vi "UHR-Fleezers Control (host) - 12.3.1.vi"() -> ()   [LabVIEW 2012] (continued)
              }
            }
          }
          frame #3 {
            n739 = property on="Sample Channel\nFlow" class="Bool (strict)"("Val(Sgnl)"=FALSE ("Value (Signaling)")) -> ()  [unwired: 2 in, 2 out]
            n740 = case shown="False" "Cap. 2 BD T1?\n(ADig T1, DNA T2)" {
              tunnel: "Cap 2 T ON" -> [w1060 w1061]
              frame False {
                n741 = property on="Trap 2 (ON/OFF)" class="Bool (strict)"("Val(Sgnl)"=w1060) -> ()  [unwired: 2 in, 2 out]
              }
              frame True {
                n742 = property on="Trap 1 (ON/OFF)" class="Bool (strict)"("Val(Sgnl)"=w1061) -> ()  [unwired: 2 in, 2 out]
              }
            }
            n743 = property on="Got ADig bead" class="Bool"("Key Focus"=TRUE) -> ()  [unwired: 2 in, 2 out]
          }
        }
      }
      event "Read Harvard": Value Change {
        n744 = event-data() -> ()  [unwired: 1 in, 5 out]
        n745 = Concatenate Strings("write buffer", "\r") -> (w1066:string)
        n746 = VISA Write(VISA resource name=w1064, write buffer=w1066, error in (no error)=w1063) -> (VISA resource name out=w1075:refnum<visa-resource-name>, error out=w1074:errorcluster)  [unwired: 1 out]
        n747 = stacked-sequence {
          tunnel: [w1078] -> w1073
          tunnel: w1075 -> [w1078]
          tunnel: w1074 -> [w1077]
          tunnel: [w1077] -> w1068
          frame #0 {
            n748 = Wait (ms)(milliseconds to wait=50) -> ()  [unwired: 1 out]
          }
        }
        n749 = property class="Instr"(reference=w1073, error in=w1068) -> (reference out=w1072:refnum<visa-resource-name>, error out=w1070:errorcluster, "Serial Settings:Number of Bytes at Serial Port"=w1071:u32)
        "Serial Settings:Number of Bytes at Serial Port" <- w1071
        n750 = VISA Read(VISA resource name=w1072, byte count=w1071, error in (no error)=w1070) -> (read buffer=w1069:string)  [unwired: 3 out]
        "read buffer" <- w1069
        n751 = Fract/Exp String To Number(string=w1069) -> ()  [unwired: 5 out]
      }
      event "+z", "-z": Value Change {
        n752 = event-data() -> ()  [unwired: 1 in, 5 out]
        n753 = flat-sequence {
          tunnel: w1079 -> [w1101]
          tunnel: w1080 -> [w1081]
          frame #0 {
            n754 = call "Read Stage Position.vi"("error in"=w1101, "VISA resource name in"=w1081) -> ("Current Position"=w1086:cluster{dbl, dbl, dbl}, "error out"=w1099:errorcluster, "VISA resource name out"=w1100:refnum<visa-resource-name>)  [unwired: 1 out]
            n755 = local read "Saved Stage Positions"() -> (w1110:dbl[][])
            n756 = Divide(x="z nudge increment (um)", y=1000.0) -> (x/y=w1098:dbl)
            n757 = Boolean To (0,1)(Boolean="+z") -> (0, 1=w1090:i16)
            n758 = Boolean To (0,1)(Boolean="-z") -> (0, 1=w1091:i16)
            n759 = Array Subset(array=w1110, index (row)=1 ("index"), length (row)=1 ("length"), index (col)=1 ("index"), length (col)=3 ("length")) -> (w1107:dbl[][])
            n760 = Multiply(x=w1090, y=w1098) -> (x*y=w1094:dbl)
            n761 = Multiply(x=w1091, y=w1098) -> (x*y=w1092:dbl)
            n762 = Unbundle(w1086) -> (w1084:dbl, w1083:dbl, w1087:dbl)
            n763 = Negate(x=w1092) -> (-x=w1093:dbl)
            n764 = Reshape Array(w1107, 3 ("dimension size")) -> (w1105:dbl[])
            n765 = Add(x=w1094, y=w1093) -> (x+y=w1095:dbl)
            n766 = Array To Cluster(array=w1105) -> ()  [unwired: 1 out]
            n767 = Add(x=w1095, y=w1087) -> (x+y=w1085:dbl)
            n768 = Bundle(cluster=w1086, w1084, w1083, w1085) -> (w1082:cluster{dbl, dbl, dbl})
            n769 = call "Set Stage Position.vi"("Position"=w1082, "error in"=w1099, "VISA resource name in"=w1100) -> ("error out"=w1104:errorcluster)  [unwired: 2 out]
            n770 = local write "Stage Moving"(TRUE ("Stage Moving")) -> ()
            n771 = local write "Stage Control Serial Error"(w1104) -> ()
          }
          frame #1 {
            n772 = local write "Stage Moving"(FALSE ("Stage Moving")) -> ()
            n773 = call <vilib>:"Beep.vi"() -> ()  [unwired: 3 in, 9 out]
          }
        }
      }
      event "Cal/Data Acq. Spot": Value Change {
        n774 = event-data() -> ()  [unwired: 1 in, 5 out]
        n775 = flat-sequence {
          tunnel: w1119 -> [w1123]
          tunnel: w1120 -> [w1124]
          tunnel: [w1124] -> w1116
          tunnel: [w1123] -> w1115
          tunnel: w1116 -> [w1129]
          tunnel: w1115 -> [w1128]
          tunnel: ["Cal @ (MHz)"] -> w1113
          tunnel: [w1133] -> w1117
          tunnel: w1113 -> [w1133]
          tunnel: w1117 -> [w1142]
          tunnel: ["W/ Offset 1"] -> w1114
          tunnel: w1117 -> [w1163]
          tunnel: w1114 -> [w1161]
          frame #0 {
            n776 = property on="Sample Channel\nFlow" class="Bool (strict)"("Val(Sgnl)"="Daq spot flow on") -> ()  [unwired: 2 in, 2 out]
            n777 = Wait (ms)(milliseconds to wait=u32 250) -> ()  [unwired: 1 out]
          }
          frame #1 {
            n778 = local read "Saved Stage Positions"() -> (w1126:dbl[][])
            n779 = property on="Trap Delta (MHz)" class="DigNum (strict)"("Val(Sgnl)"="Cal @ (MHz)") -> ()  [unwired: 2 in, 2 out]
            n780 = local write "Stage Moving"(TRUE ("Stage Moving")) -> ()
            n781 = call "move to saved stage position.vi"("error in"=w1128, "Stage VISA resource name in"=w1129, "Position"="Cal Stage Position", "Saved Stage Positions"=w1126) -> ("error out"=w1127:errorcluster)  [unwired: 1 out]
            n782 = local write "Stage Control Serial Error"(w1127) -> ()
          }
          frame #2 {
            n783 = local write "Stage Moving"(FALSE ("Stage Moving")) -> ()
            n784 = property on="Sample Channel\nFlow" class="Bool (strict)"("Val(Sgnl)"="Flow ON during cal?") -> ()  [unwired: 2 in, 2 out]
            n785 = call <vilib>:"Beep.vi"() -> ()  [unwired: 3 in, 9 out]
          }
          frame #3 {
            n786 = Wait (ms)(milliseconds to wait=u32 1000) -> ()  [unwired: 1 out]
          }
          frame #4 {
            n787 = property on="Save Calibration" class="Bool (strict)"("Val(Sgnl)"=TRUE ("Value (Signaling)")) -> ()  [unwired: 2 in, 2 out]
          }
          frame #5 {
            n788 = Wait (ms)(milliseconds to wait=u32 2000) -> ()  [unwired: 1 out]
          }
          frame #6 {
            # "Check to see if \nsaving done"
            n789 = while {
              stop <- w1138 stop-if-true
              n790 = local read "Saving..."() -> (w1139:bool)
              n791 = Wait (ms)(milliseconds to wait=u32 100) -> ()  [unwired: 1 out]
              n792 = Not(x=w1139) -> (.not. x?=w1138:bool)
            }
          }
          frame #7 {
            n793 = case shown="True" "W/ Offset 1" {
              tunnel: w1142 -> [_ w1143]
              frame False {
              }
              frame True {
                n794 = stacked-sequence {
                  tunnel: w1143 -> [_ _ _ _ _ _ _ w1160]
                  frame #0 {
                    n795 = property on="Trap Delta (MHz)" class="DigNum (strict)"("Val(Sgnl)"="Offset 1 Start (MHz)") -> ()  [unwired: 2 in, 2 out]
                    n796 = Replace Array Subset(array=u32[] [0] ("Index Values"), new element="Offset 1 Set", index=0) -> (w1144:u32[])
                    n797 = property on="Saved AOD Raster Scan Parameter Sets" class="Arr (strict)"("Index Values"=w1144) -> ()  [unwired: 2 in, 2 out]
                  }
                  frame #1 {
                    n798 = Wait (ms)(milliseconds to wait=u32 200) -> ()  [unwired: 1 out]
                  }
                  frame #2 {
                    n799 = property on="Load parameters" class="Bool (strict)"("Val(Sgnl)"=TRUE ("Value (Signaling)")) -> ()  [unwired: 2 in, 2 out]
                  }
                  frame #3 {
                    n800 = Wait (ms)(milliseconds to wait=u32 200) -> ()  [unwired: 1 out]
                  }
                  frame #4 {
                    n801 = property on="Trap Raster Scan" class="Bool (strict)"("Val(Sgnl)"=TRUE ("Value (Signaling)")) -> ()  [unwired: 2 in, 2 out]
                  }
                  frame #5 {
                    n802 = Wait (ms)(milliseconds to wait=u32 2000) -> ()  [unwired: 1 out]
                  }
                  frame #6 {
                    n803 = while {
                      stop <- w1157 stop-if-true
                      n804 = local read "Raster Scanning..."() -> (w1159:bool)
                      n805 = local read "Saving..."() -> (w1155:bool)
                      n806 = Wait (ms)(milliseconds to wait=u32 100) -> ()  [unwired: 1 out]
                      n807 = Not(x=w1155) -> (.not. x?=w1154:bool)
                      n808 = Not(x=w1159) -> (.not. x?=w1156:bool)
                      n809 = And(x=w1156, y=w1154) -> (x .and. y?=w1157:bool)
                    }
                  }
                  frame #7 {
                    n810 = property on="Trap Delta (MHz)" class="DigNum (strict)"("Val(Sgnl)"=w1160) -> ()  [unwired: 2 in, 2 out]
                  }
                }
              }
            }
          }
          frame #8 {
            n811 = local read "Save ave N"() -> (w1162:dbl)
            n812 = case shown="False" "W/ Offset 2" {
              tunnel: w1163 -> [_ w1170]
              tunnel: w1162 -> [_ w1169]
              tunnel: w1161 -> [w1165 _]
              frame False {
                n813 = case shown="False" w1165 {
                  frame False {
                    n814 = Multiply(x="Cal read wait (s)", y=u32 1000 ("milliseconds to wait")) -> (x*y=w1167:u32)
                    n815 = Wait (ms)(milliseconds to wait=w1167) -> ()  [unwired: 1 out]
                  }
                  frame True {
                  }
                }
              }
              frame True {
                n816 = stacked-sequence {
                  tunnel: w1170 -> [_ _ _ _ _ _ _ _ _ w1191 _ _]
                  tunnel: w1169 -> [_ _ _ _ _ _ _ _ _ w1189 _ _]
                  frame #0 {
                    n817 = property on="Save ave N" class="DigNum (strict)"("Val(Sgnl)"=1.0 ("Value (Signaling)")) -> ()  [unwired: 2 in, 2 out]
                  }
                  frame #1 {
                    n818 = Wait (ms)(milliseconds to wait=u32 500) -> ()  [unwired: 1 out]
                  }
                  frame #2 {
                    n819 = property on="Trap Delta (MHz)" class="DigNum (strict)"("Val(Sgnl)"="Offset 2 Start (MHz)") -> ()  [unwired: 2 in, 2 out]
                    n820 = Replace Array Subset(array=u32[] [0] ("Index Values"), new element="Offset 2 Set", index=0) -> (w1175:u32[])
                    n821 = property on="Saved AOD Raster Scan Parameter Sets" class="Arr (strict)"("Index Values"=w1175) -> ()  [unwired: 2 in, 2 out]
                  }
                  frame #3 {
                    n822 = Wait (ms)(milliseconds to wait=u32 500) -> ()  [unwired: 1 out]
                  }
                  frame #4 {
                    n823 = property on="Load parameters" class="Bool (strict)"("Val(Sgnl)"=TRUE ("Value (Signaling)")) -> ()  [unwired: 2 in, 2 out]
                  }
                  frame #5 {
                    n824 = Wait (ms)(milliseconds to wait=u32 500) -> ()  [unwired: 1 out]
                  }
                  frame #6 {
                    n825 = property on="Trap Raster Scan" class="Bool (strict)"("Val(Sgnl)"=TRUE ("Value (Signaling)")) -> ()  [unwired: 2 in, 2 out]
                  }
                  frame #7 {
                    n826 = Wait (ms)(milliseconds to wait=u32 2000) -> ()  [unwired: 1 out]
                  }
                  frame #8 {
                    n827 = while {
                      stop <- w1184 stop-if-true
                      n828 = local read "Raster Scanning..."() -> (w1187:bool)
                      n829 = local read "Saving..."() -> (w1185:bool)
                      n830 = Wait (ms)(milliseconds to wait=u32 100) -> ()  [unwired: 1 out]
                      n831 = Not(x=w1185) -> (.not. x?=w1183:bool)
                      n832 = Not(x=w1187) -> (.not. x?=w1186:bool)
                      n833 = And(x=w1186, y=w1183) -> (x .and. y?=w1184:bool)
                    }
                  }
                  frame #9 {
                    n834 = property on="Trap Delta (MHz)" class="DigNum (strict)"("Val(Sgnl)"=w1191) -> ()  [unwired: 2 in, 2 out]
                    n835 = property on="Saved AOD Raster Scan Parameter Sets" class="Arr (strict)"("Index Values"=u32[] [0]) -> ()  [unwired: 2 in, 2 out]
                    n836 = property on="Save ave N" class="DigNum (strict)"("Val(Sgnl)"=w1189) -> ()  [unwired: 2 in, 2 out]
                  }
                  frame #10 {
                    n837 = Wait (ms)(milliseconds to wait=u32 500) -> ()  [unwired: 1 out]
                  }
                  frame #11 {
                    n838 = property on="Load parameters" class="Bool (strict)"("Val(Sgnl)"=TRUE ("Value (Signaling)")) -> ()  [unwired: 2 in, 2 out]
                  }
                }
              }
            }
          }
          frame #9 {
            n839 = property on="Read Cal" class="Bool (strict)"("Val(Sgnl)"=TRUE ("Value (Signaling)")) -> ()  [unwired: 2 in, 2 out]
          }
          frame #10 {
            n840 = Wait (ms)(milliseconds to wait=u32 1000) -> ()  [unwired: 1 out]
          }
          frame #11 {
            n841 = property on="Fish for Tether" class="Bool (strict)"("Val(Sgnl)"=TRUE ("Value (Signaling)")) -> ()  [unwired: 2 in, 2 out]
          }
        }
        n842 = local write "Cal/Data Acq. Spot"(FALSE ("Cal/Data Acq. Spot")) -> ()
      }
      event "Dump Beads": Value Change {
        n843 = event-data() -> ()  [unwired: 1 in, 5 out]
        n844 = flat-sequence {
          tunnel: ["Dump spot flow on?"] -> w1197
          tunnel: [w1208] -> w1198
          tunnel: w1197 -> [w1208]
          tunnel: w1201 -> [w1213]
          tunnel: w1200 -> [w1212]
          tunnel: [w1210] -> w1199
          tunnel: w1198 -> [w1210]
          tunnel: w1199 -> [w1223]
          frame #0 {
            w1202 = FALSE ("Value (Signaling)")
            n845 = local read "Saving..."() -> (w1204:bool)
            n846 = local write "Dump Beads"(FALSE ("Dump Beads")) -> ()
            n847 = property on="Inject Pump 3" class="Bool (strict)"("Val(Sgnl)"=w1202) -> ()  [unwired: 2 in, 2 out]
            n848 = property on="Inject Pump 1" class="Bool (strict)"("Val(Sgnl)"=w1202) -> ()  [unwired: 2 in, 2 out]
            n849 = local write "Stop Saving"(w1204) -> ()
          }
          frame #1 {
            w1205 = FALSE ("Fl. Triggered...")
            n850 = case shown="True" "Dump spot flow on?" {
              frame False {
              }
              frame True {
                n851 = property on="Sample Channel\nFlow" class="Bool (strict)"("Val(Sgnl)"=TRUE ("Stage Moving")) -> ()  [unwired: 2 in, 2 out]
              }
            }
            n852 = local write "Fl. Triggered..."(w1205) -> ()
            n853 = local write "Tether"(w1205) -> ()
            n854 = property on="Green Laser ON" class="Bool (strict)"("Val(Sgnl)"=w1205) -> ()  [unwired: 2 in, 2 out]
            n855 = property on="Trap Pos. FB ON" class="Bool (strict)"("Val(Sgnl)"=w1205) -> ()  [unwired: 2 in, 2 out]
            n856 = property on="Trap Trig. Fl." class="Bool (strict)"("Val(Sgnl)"=w1205) -> ()  [unwired: 2 in, 2 out]
            n857 = property on="Fl. Triggered..." class="Bool (strict)"("Val(Sgnl)"=w1205) -> ()  [unwired: 2 in, 2 out]
            n858 = property on="Dip for Protein" class="Bool (strict)"("Val(Sgnl)"=w1205) -> ()  [unwired: 2 in, 2 out]
            n859 = property on="Pause dwell" class="Bool (strict)"("Val(Sgnl)"=w1205) -> ()  [unwired: 2 in, 2 out]
          }
          frame #2 {
            n860 = property on="Trap Pos. FB Offset Factor" class="DigNum (strict)"("Val(Sgnl)"=i64 0 ("Value (Signaling)")) -> ()  [unwired: 2 in, 2 out]
          }
          frame #3 {
            n861 = local read "Saved Stage Positions"() -> (w1214:dbl[][])
            n862 = local write "Stage Moving"(TRUE ("Stage Moving")) -> ()
            n863 = Array Subset(array=w1214, index (row)=3 ("index"), length (row)=1 ("length"), index (col)=1 ("index"), length (col)=3 ("length")) -> (w1219:dbl[][])
            n864 = Reshape Array(w1219, 3 ("dimension size")) -> (w1217:dbl[])
            n865 = Array To Cluster(array=w1217) -> (cluster=w1216:cluster{"[0]":dbl, "[1]":dbl, "[2]":dbl})
            n866 = call "Set Stage Position.vi"("Position"=w1216, "error in"=w1212, "VISA resource name in"=w1213) -> ()  [unwired: 3 out]
          }
          frame #4 {
            w1224 = FALSE ("Value (Signaling)")
            n867 = case shown="True" w1223 {
              frame False {
              }
              frame True {
                n868 = property on="Sample Channel\nFlow" class="Bool (strict)"("Val(Sgnl)"=FALSE ("Stage Moving")) -> ()  [unwired: 2 in, 2 out]
              }
            }
            n869 = property on="Trap 1 (ON/OFF)" class="Bool (strict)"("Val(Sgnl)"=w1224) -> ()  [unwired: 2 in, 2 out]
            n870 = property on="Trap 2 (ON/OFF)" class="Bool (strict)"("Val(Sgnl)"=w1224) -> ()  [unwired: 2 in, 2 out]
            n871 = call <vilib>:"Beep.vi"() -> ()  [unwired: 3 in, 9 out]
          }
          frame #5 {
            n872 = property on="Move Cap. 2 (ADig Top)" class="Bool (strict)"("Val(Sgnl)"=TRUE ("Value (Signaling)")) -> ()  [unwired: 2 in, 2 out]
            n873 = property on="Tab Control" class="TabCtl (strict)"("Val(Sgnl)"=T24."Status" ("Value (Signaling)")) -> ()  [unwired: 2 in, 2 out]
          }
        }
      }
      event "Dip for Protein": Value Change {
        n874 = event-data() -> ()  [unwired: 1 in, 5 out]
        n875 = case shown="True" "Dip for Protein" {
          tunnel: w1230 -> [_ w1232]
          tunnel: w1229 -> [_ w1231]
          frame False {
          }
          frame True {
            n876 = while {
              tunnel: w1232 -> [w1243]
              tunnel: w1231 -> [w1242]
              i -> [w1237]
              stop <- w1239 stop-if-true
              n877 = Increment(x=w1237) -> (x+1=→"Dip #":i32)
              n878 = flat-sequence {
                tunnel: w1242 -> [w1254]
                tunnel: w1243 -> [w1255]
                tunnel: [w1255] -> w1247
                tunnel: [w1254] -> w1246
                tunnel: [w1248] -> w1233
                tunnel: [w1260] -> w1241
                tunnel: [w1261] -> w1240
                tunnel: w1247 -> [w1262]
                tunnel: w1246 -> [w1263]
                tunnel: [w1258] -> w1234
                tunnel: w1233 -> [w1258]
                tunnel: [w1271] -> w1245
                tunnel: w1241 -> [w1271]
                tunnel: [w1270] -> w1244
                tunnel: w1240 -> [w1270]
                tunnel: [w1267] -> w1238
                tunnel: [w1266] -> w1235
                tunnel: w1234 -> [w1266]
                tunnel: w1244 -> [w1291]
                tunnel: w1245 -> [w1292]
                tunnel: w1238 -> [w1293]
                tunnel: w1235 -> [w1290]
                tunnel: [w1349] -> w1239
                frame #0 {
                  n879 = local read "Trap Pos. FB ON"() -> (w1248:bool)
                  n880 = Compound Arithmetic op=AND("Flow ON\nduring dip?", "FB OFF when \nflow ON", w1248) -> (w1249:bool)
                  n881 = case shown="True" "Move trap \nbefore dip move?" {
                    frame False {
                    }
                    frame True {
                      n882 = property on="Trap Delta (MHz)" class="DigNum (strict)"("Val(Sgnl)"="Dipping Delta (MHz)") -> ()  [unwired: 2 in, 2 out]
                    }
                  }
                  n883 = property on="Green Laser ON" class="Bool (strict)"("Val(Sgnl)"="Green ON\nbefore dip?") -> ()  [unwired: 2 in, 2 out]
                  n884 = property on="Sample Channel\nFlow" class="Bool (strict)"("Val(Sgnl)"="Flow ON\nduring dip?") -> ()  [unwired: 2 in, 2 out]
                  n885 = case shown="True" w1249 {
                    frame False {
                    }
                    frame True {
                      n886 = property on="Trap Pos. FB ON" class="Bool (strict)"("Val(Sgnl)"=FALSE ("Value (Signaling)")) -> ()  [unwired: 2 in, 2 out]
                    }
                  }
                }
                frame #1 {
                  n887 = local read "Saved Stage Positions"() -> (w1265:dbl[][])
                  n888 = local write "Cancel dwell"(FALSE ("Cancel dwell")) -> ()
                  n889 = call "move to saved stage position.vi"("error in"=w1263, "Stage VISA resource name in"=w1262, "Position"="Dip Stage \nPosition", "Saved Stage Positions"=w1265) -> ("VISA resource name out"=w1260:refnum<visa-resource-name>, "error out"=w1261:errorcluster)
                }
                frame #2 {
                  n890 = node-c288() -> (w1269:T21)  [unwired: 4 in]
                  n891 = timed-loop {
                    timing: w1269 -> [_]
                    timing-out: [_] -> w1268
                    tunnel: [w1275] -> w1267
                    i -> [w1272]
                    stop <- w1276 stop-if-true
                    n892 = node-c288() -> ()  [unwired: 1 in, 1 out]
                    n893 = Greater Or Equal?(x=w1272, y="Dip Duration (s)") -> (x >= y?=w1284:bool)
                    n894 = local read "Dip for Protein"() -> (w1277:bool)
                    n895 = local read "Dump Beads"() -> (w1274:bool)
                    n896 = local read "Cancel dwell"() -> (w1283:bool)
                    n897 = local read "Pause dwell"() -> (w1280:bool)
                    n898 = Not(x=w1277) -> (.not. x?=w1282:bool)
                    n899 = Compound Arithmetic op=OR(w1283, w1284, w1282) -> (w1281:bool)
                    n900 = Select(t=FALSE, s=w1280, f=w1281) -> (s? t:f=w1278:bool)
                    n901 = Not(x=w1274) -> (.not. x?=w1273:bool)
                    n902 = node-c288() -> ()  [unwired: 1 in, 1 out]
                    n903 = And(x=w1277, y=w1273) -> (x .and. y?=w1275:bool)
                    n904 = Or(x=w1278, y=w1274) -> (x .or. y?=w1276:bool)
                    "Dip Time (s)" <- w1272
                  }
                  n905 = node-c288(w1268) -> ()  [unwired: 1 out]
                }
                frame #3 {
                  n906 = case shown="True" w1293 {
                    tunnel: w1292 -> [_ w1298]
                    tunnel: w1291 -> [_ w1297]
                    tunnel: w1290 -> [_ w1294]
                    frame False {
                    }
                    frame True {
                      n907 = flat-sequence {
                        tunnel: w1297 -> [w1302]
                        tunnel: w1298 -> [w1303]
                        tunnel: [w1303] -> w1296
                        tunnel: [w1302] -> w1295
                        tunnel: w1294 -> [w1299]
                        tunnel: w1296 -> [w1313]
                        tunnel: w1295 -> [w1312]
                        tunnel: w1294 -> [w1321]
                        frame #0 {
                          n908 = local read "Sample Channel\nFlow"() -> (w1301:bool)
                          n909 = case shown="True" w1301 {
                            tunnel: "Flow ON \nduring return\nfrom dip?" -> [w1304 w1307]
                            tunnel: w1299 -> [_ w1306]
                            frame False {
                              n910 = case shown="True" w1304 {
                                frame False {
                                }
                                frame True {
                                n911 = property on="Sample Channel\nFlow" class="Bool (strict)"("Val(Sgnl)"=TRUE ("Value (Signaling)")) -> ()  [unwired: 2 in, 2 out]
                                }
                              }
                            }
                            frame True {
                              n912 = case shown="False" w1307 {
                                tunnel: w1306 -> [w1308 _]
                                frame False {
                                n913 = property on="Trap Pos. FB ON" class="Bool (strict)"("Val(Sgnl)"=w1308) -> ()  [unwired: 2 in, 2 out]
                                n914 = property on="Sample Channel\nFlow" class="Bool (strict)"("Val(Sgnl)"=FALSE ("Value (Signaling)")) -> ()  [unwired: 2 in, 2 out]
                                }
                                frame True {
                                }
                              }
                            }
                          }
                        }
                        frame #1 {
                          # "For turning on green laser before stage reaches lower spot"
                          n915 = case shown="True" "Green ON\nafter start\nreturn?" {
                            frame False {
                            }
                            frame True {
                              n916 = flat-sequence {
                                frame #0 {
                                n917 = Multiply(x="Green delay after \nstart return (s)", y=1000.0) -> (x*y=w1318:dbl)
                                n918 = Wait (ms)(milliseconds to wait=w1318) -> ()  [unwired: 1 out]
                                }
                                frame #1 {
                                n919 = property on="Green Laser ON" class="Bool (strict)"("Val(Sgnl)"=TRUE ("Value (Signaling)")) -> ()  [unwired: 2 in, 2 out]
                                }
                              }
                            }
                          }
                          n920 = local read "Saved Stage Positions"() -> (w1316:dbl[][])
                          n921 = local write "Cancel dwell"(FALSE ("Cancel dwell")) -> ()
                          n922 = call "move to saved stage position.vi"("error in"=w1312, "Stage VISA resource name in"=w1313, "Position"="Return Stage \nPosition", "Saved Stage Positions"=w1316) -> ("error out"=w1314:errorcluster)  [unwired: 1 out]
                          n923 = local write "Stage Control Serial Error"(w1314) -> ()
                        }
                        frame #2 {
                          n924 = property on="Trap Pos. FB ON" class="Bool (strict)"("Val(Sgnl)"=w1321) -> ()  [unwired: 2 in, 2 out]
                          n925 = case shown="True" "Green ON \nafter return?" {
                            frame False {
                            }
                            frame True {
                              n926 = property on="Green Laser ON" class="Bool (strict)"("Val(Sgnl)"=TRUE ("Value (Signaling)")) -> ()  [unwired: 2 in, 2 out]
                            }
                          }
                          n927 = case shown="True" "Move trap after return?" {
                            frame False {
                            }
                            frame True {
                              n928 = property on="Trap Delta (MHz)" class="DigNum (strict)"("Val(Sgnl)"="Dip Trap Delta 2 (MHz)") -> ()  [unwired: 2 in, 2 out]
                            }
                          }
                          n929 = case shown="True" "Save data after return?" {
                            frame False {
                            }
                            frame True {
                              n930 = property on="Start Saving" class="Bool (strict)"("Val(Sgnl)"=TRUE ("Value (Signaling)")) -> ()  [unwired: 2 in, 2 out]
                            }
                          }
                          n931 = property on="Sample Channel\nFlow" class="Bool (strict)"("Val(Sgnl)"="Flow ON\nduring daq?") -> ()  [unwired: 2 in, 2 out]
                        }
                        frame #3 {
                          n932 = node-c288() -> (w1330:T21)  [unwired: 4 in]
                          n933 = timed-loop {
                            timing: w1330 -> [_]
                            timing-out: [_] -> w1329
                            i -> [w1331]
                            stop <- w1333 stop-if-true
                            n934 = node-c288() -> ()  [unwired: 1 in, 1 out]
                            n935 = local read "Dump Beads"() -> (w1332:bool)
                            n936 = Greater Or Equal?(x=w1331, y="Dwell Duration (s)") -> (x >= y?=w1338:bool)
                            n937 = local read "Dip for Protein"() -> (w1335:bool)
                            n938 = Not(x=w1335) -> (.not. x?=w1334:bool)
                            n939 = Compound Arithmetic op=OR(w1338, "Cancel dwell", w1334) -> (w1337:bool)
                            n940 = node-c288() -> ()  [unwired: 1 in, 1 out]
                            n941 = Select(t=FALSE, s="Pause dwell", f=w1337) -> (s? t:f=w1340:bool)
                            n942 = Or(x=w1340, y=w1332) -> (x .or. y?=w1333:bool)
                            "Dwell Time (s)" <- w1331
                          }
                          n943 = node-c288(w1329) -> ()  [unwired: 1 out]
                        }
                      }
                    }
                  }
                }
                frame #4 {
                  n944 = local read "Dip for Protein"() -> (w1350:bool)
                  n945 = local read "Dump Beads"() -> (w1347:bool)
                  n946 = local write "Cancel dwell"(FALSE ("Cancel dwell")) -> ()
                  n947 = Not(x=w1350) -> (.not. x?=w1351:bool)
                  n948 = Not(x="Cont. Repeat Dipping?") -> (.not. x?=w1353:bool)
                  n949 = Compound Arithmetic op=OR(w1351, w1353, w1347) -> (w1349:bool)
                }
              }
            }
          }
        }
      }
      event "Profile": Value Change {
        n950 = event-data() -> ()  [unwired: 1 in, 5 out]
        n951 = flat-sequence {
          tunnel: w1362 -> [w1365]
          tunnel: w1361 -> [w1373]
          tunnel: [w1367] -> w1360
          tunnel: [w1366] -> w1359
          tunnel: [w1364] -> w1357
          tunnel: [w1363] -> w1354
          tunnel: w1360 -> [w1380]
          tunnel: w1359 -> [w1379]
          tunnel: [w1377] -> w1358
          tunnel: w1357 -> [w1378]
          tunnel: [w1376] -> w1356
          tunnel: [w1375] -> w1355
          tunnel: w1354 -> [w1375]
          tunnel: w1358 -> [w1384]
          tunnel: w1356 -> [w1383]
          tunnel: w1355 -> [w1382]
          frame #0 {
            n952 = call "Read Stage Position.vi"("error in"=w1373, "VISA resource name in"=w1365) -> ("Current Position"=w1363:cluster{dbl, dbl, dbl}, "error out"=w1366:errorcluster, "VISA resource name out"=w1364:refnum<visa-resource-name>)  [unwired: 1 out]
            "Current Position" <- w1363
            n953 = local write "Stage Control Serial Error"(w1366) -> ()
            n954 = Unbundle(w1363) -> (w1370:dbl, w1372:dbl, w1368:dbl)
            n955 = Add(x=w1372, y="Y change (mm)") -> (x+y=w1369:dbl)
            n956 = Bundle(w1370, w1369, w1368) -> (w1367:cluster{dbl, dbl, dbl})  [unwired: 1 in]
          }
          frame #1 {
            # "move to new position and start saving"
            n957 = local write "Stage Moving"(TRUE ("Stage Moving")) -> ()
            n958 = local write "Start Saving"(TRUE ("Start Saving")) -> ()
            n959 = call "Set Stage Position.vi"("Position"=w1380, "error in"=w1379, "VISA resource name in"=w1378) -> ("error out"=w1376:errorcluster, "VISA resource name out"=w1377:refnum<visa-resource-name>)  [unwired: 1 out]
          }
          frame #2 {
            # "go back to start"
            n960 = call "Set Stage Position.vi"("Position"=w1382, "error in"=w1383, "VISA resource name in"=w1384) -> ()  [unwired: 3 out]
          }
          frame #3 {
            # "stop saving"
            n961 = local write "Stop Saving"(TRUE ("Stop Saving")) -> ()
            n962 = local write "Stage Moving"(FALSE ("Stage Moving")) -> ()
          }
        }
      }
      event "Move to Position 1", "Move to Position 2", "Move to Position 3", "Move to Position 4", "Move to Position 5", "Lower Ch. Cap.": Value Change {
        n963 = event-data() -> ()  [unwired: 1 in, 5 out]
        n964 = Or(x="Move to Position 5", y="Lower Ch. Cap.") -> (x .or. y?=w1390:bool)
        n965 = Build Array("Move to Position 1", "Move to Position 2", "Move to Position 3", "Move to Position 4", w1390) -> (w1393:bool[])
        n966 = Boolean Array To Number(Boolean array=w1393) -> (number=w1392:u32)
        n967 = Logarithm Base 2(1:w1392) -> (0:w1391:dbl)
        n968 = flat-sequence {
          tunnel: w1391 -> [w1402]
          tunnel: w1388 -> [w1400]
          tunnel: w1387 -> [w1399]
          frame #0 {
            n969 = local read "Saved Stage Positions"() -> (w1410:dbl[][])
            n970 = Array Subset(array=w1410, index (row)=w1402, length (row)=1 ("length"), index (col)=1 ("index"), length (col)=3 ("length")) -> (w1407:dbl[][])
            n971 = Reshape Array(w1407, 3 ("dimension size")) -> (w1405:dbl[])
            n972 = Array To Cluster(array=w1405) -> (cluster=w1404:cluster{"[0]":dbl, "[1]":dbl, "[2]":dbl})
            n973 = call "Set Stage Position.vi"("Position"=w1404, "error in"=w1399, "VISA resource name in"=w1400) -> ("error out"=w1403:errorcluster)  [unwired: 2 out]
            n974 = local write "Stage Moving"(TRUE ("Stage Moving")) -> ()
            n975 = local write "Stage Control Serial Error"(w1403) -> ()
          }
          frame #1 {
            n976 = local write "Stage Moving"(FALSE ("Stage Moving")) -> ()
            n977 = call <vilib>:"Beep.vi"() -> ()  [unwired: 3 in, 9 out]
          }
        }
      }
      event "Got ADig bead": Value Change {
        n978 = event-data() -> ()  [unwired: 1 in, 5 out]
        n979 = flat-sequence {
          frame #0 {
            n980 = local read "Cap 1 Samp Flow ON"() -> (w1414:bool)
            n981 = case shown="True" w1414 {
              frame False {
              }
              frame True {
                n982 = property on="Sample Channel\nFlow" class="Bool (strict)"("Val(Sgnl)"=TRUE ("Value (Signaling)")) -> ()  [unwired: 2 in, 2 out]
              }
            }
          }
          frame #1 {
            n983 = property on="Inject Pump 3" class="Bool (strict)"("Val(Sgnl)"=FALSE ("Value (Signaling)")) -> ()  [unwired: 2 in, 2 out]
          }
          frame #2 {
            n984 = property on="Move Cap. 1 (DNA Bottom)" class="Bool (strict)"("Val(Sgnl)"=TRUE ("Value (Signaling)")) -> ()  [unwired: 2 in, 2 out]
          }
        }
      }
      event "Force FB Data\nScript": Value Change {
        n985 = event-data() -> ()  [unwired: 1 in, 5 out]
        n986 = flat-sequence {
          tunnel: w1423 -> [w1427]
          tunnel: w1424 -> [w1428]
          tunnel: [w1428] -> w1419
          tunnel: [w1427] -> w1418
          tunnel: w1419 -> [w1431]
          tunnel: w1418 -> [w1430]
          tunnel: ["Trap Trig Fl."] -> w1420
          tunnel: [w1456] -> w1421
          tunnel: w1420 -> [w1456]
          tunnel: [w1460] -> w1422
          tunnel: w1421 -> [w1460]
          tunnel: w1422 -> [w1462]
          frame #0 {
            n987 = property on="Trap Delta (MHz)" class="DigNum (strict)"("Val(Sgnl)"="Trap Delta Before Moving") -> ()  [unwired: 2 in, 2 out]
          }
          frame #1 {
            n988 = local read "Saved Stage Positions"() -> (w1433:dbl[][])
            n989 = local write "FB Trap Pos Offset"(0.0 ("FB Trap Pos Offset")) -> ()
            n990 = property on="Trap Pos. FB Offset Factor" class="DigNum (strict)"("Val(Sgnl)"=i64 0 ("Value (Signaling)")) -> ()  [unwired: 2 in, 2 out]
            n991 = local write "Stage Moving"(TRUE ("Stage Moving")) -> ()
            n992 = call "move to saved stage position.vi"("error in"=w1430, "Stage VISA resource name in"=w1431, "Position"="Stage Position To Establish FB", "Saved Stage Positions"=w1433) -> ("error out"=w1429:errorcluster)  [unwired: 1 out]
            n993 = local write "Stage Control Serial Error"(w1429) -> ()
          }
          frame #2 {
            n994 = call <vilib>:"Beep.vi"() -> ()  [unwired: 3 in, 9 out]
            n995 = Multiply(x="Wait (s)", y=u32 1000 ("milliseconds to wait")) -> (x*y=w1440:u32)
            n996 = property on="Trap Delta (MHz)" class="DigNum (strict)"("Val(Sgnl)"="Starting \nTrap Delta (MHz)") -> ()  [unwired: 2 in, 2 out]
            n997 = local write "Stage Moving"(FALSE ("Stage Moving")) -> ()
            n998 = Wait (ms)(milliseconds to wait=w1440) -> ()  [unwired: 1 out]
            n999 = property on="Tab Control 2" class="TabCtl (strict)"("Val(Sgnl)"=T6."Feedback on Trap Position" ("Value (Signaling)")) -> ()  [unwired: 2 in, 2 out]
            n1000 = property on="Tab Control" class="TabCtl (strict)"("Val(Sgnl)"=T4."Trap Control (RF)" ("Value (Signaling)")) -> ()  [unwired: 2 in, 2 out]
          }
          frame #3 {
            n1001 = property on="Set Reading to\nSetpoint" class="Bool (strict)"("Val(Sgnl)"=TRUE ("Value (Signaling)")) -> ()  [unwired: 2 in, 2 out]
            n1002 = Wait (ms)(milliseconds to wait=u32 500) -> ()  [unwired: 1 out]
          }
          frame #4 {
            n1003 = property on="Trap Pos. FB ON" class="Bool (strict)"("Val(Sgnl)"=TRUE ("Value (Signaling)")) -> ()  [unwired: 2 in, 2 out]
            n1004 = Wait (ms)(milliseconds to wait=u32 250) -> ()  [unwired: 1 out]
          }
          frame #5 {
            n1005 = case shown="False" "Trap Trig Fl." {
              frame False {
                n1006 = case shown="True" "Green ON after FB ON?" {
                  selector: "Green ON after FB ON?" -> [_ w1455]
                  frame False {
                  }
                  frame True {
                    n1007 = property on="Green Laser ON" class="Bool (strict)"("Val(Sgnl)"=w1455) -> ()  [unwired: 2 in, 2 out]
                  }
                }
              }
              frame True {
              }
            }
            n1008 = case shown="True" "Remove Action Offset" {
              tunnel: TRUE ("Value (Signaling)") -> [w1452 w1453]
              frame False {
                n1009 = property on="Remove Unwinding Offset" class="Bool (strict)"("Val(Sgnl)"=w1452) -> ()  [unwired: 2 in, 2 out]
              }
              frame True {
                n1010 = property on="Remove Action Offset" class="Bool (strict)"("Val(Sgnl)"=w1453) -> ()  [unwired: 2 in, 2 out]
              }
            }
            n1011 = Wait (ms)(milliseconds to wait=u32 250) -> ()  [unwired: 1 out]
          }
          frame #6 {
            n1012 = property on="Start Saving" class="Bool (strict)"("Val(Sgnl)"=TRUE ("Value (Signaling)")) -> ()  [unwired: 2 in, 2 out]
            n1013 = Wait (ms)(milliseconds to wait=u32 5000) -> ()  [unwired: 1 out]
          }
          frame #7 {
            w1459 = TRUE ("Value (Signaling)")
            n1014 = property on="Rem fb disp offset" class="Bool (strict)"("Val(Sgnl)"=w1459) -> ()  [unwired: 2 in, 2 out]
            n1015 = property on="Remove Offset" class="Bool (strict)"("Val(Sgnl)"=w1459) -> ()  [unwired: 2 in, 2 out]
            n1016 = Wait (ms)(milliseconds to wait=u32 100) -> ()  [unwired: 1 out]
          }
          frame #8 {
            n1017 = case shown="True" w1462 {
              frame False {
              }
              frame True {
                n1018 = local write "Trap Trig. Fl."(TRUE ("Value (Signaling)")) -> ()
              }
            }
          }
          frame #9 {
            n1019 = case shown="True" "Start dipping after?" {
              frame False {
              }
              frame True {
                n1020 = flat-sequence {
                  frame #0 {
                    n1021 = Multiply(x="Delay before dipping (s)", y=1000.0) -> (x*y=w1466:dbl)
                    n1022 = Wait (ms)(milliseconds to wait=w1466) -> ()  [unwired: 1 out]
                  }
                  frame #1 {
                    n1023 = property on="Dip for Protein" class="Bool (strict)"("Val(Sgnl)"=TRUE ("Value (Signaling)")) -> ()  [unwired: 2 in, 2 out]
                    n1024 = local write "Scripts"(T1."Dipping" ("Scripts")) -> ()
                  }
                }
              }
            }
          }
        }
      }
      event "Fixed Traps Data\nScript": Value Change {
        n1025 = event-data() -> ()  [unwired: 1 in, 5 out]
        n1026 = flat-sequence {
          frame #0 {
            n1027 = case shown="True" "Green ON" {
              frame False {
              }
              frame True {
                n1028 = property on="Green Laser ON" class="Bool (strict)"("Val(Sgnl)"=TRUE) -> ()  [unwired: 2 in, 2 out]
              }
            }
            n1029 = local write "Offset (nm)"(0.0 ("Offset (nm)")) -> ()
            n1030 = property on="Sample Channel\nFlow" class="Bool (strict)"("Val(Sgnl)"=FALSE ("Value (Signaling)")) -> ()  [unwired: 2 in, 2 out]
            n1031 = property on="Trap Delta (MHz)" class="DigNum (strict)"("Val(Sgnl)"="Fixed Traps Trap Delta (MHz)") -> ()  [unwired: 2 in, 2 out]
          }
          frame #1 {
            n1032 = Wait (ms)(milliseconds to wait=u32 1000) -> ()  [unwired: 1 out]
          }
          frame #2 {
            n1033 = local write "Start Saving"(TRUE ("Start Saving")) -> ()
          }
          frame #3 {
            n1034 = local read "Bead Sep. Int. Time (s)"() -> (w1477:dbl)
            n1035 = Multiply(x=w1477, y=1000.0) -> (x*y=w1479:dbl)
            n1036 = Wait (ms)(milliseconds to wait=w1479) -> ()  [unwired: 1 out]
          }
          frame #4 {
            n1037 = property on="Remove Offset" class="Bool (strict)"("Val(Sgnl)"=TRUE ("Value (Signaling)")) -> ()  [unwired: 2 in, 2 out]
          }
          frame #5 {
            n1038 = property on="Dip for Protein" class="Bool (strict)"("Val(Sgnl)"="Start dipping after?") -> ()  [unwired: 2 in, 2 out]
          }
        }
      }
      event "Got DNA bead": Value Change {
        n1039 = event-data() -> ()  [unwired: 1 in, 5 out]
        n1040 = flat-sequence {
          frame #0 {
            n1041 = local read "Daq spot flow on"() -> (w1484:bool)
            n1042 = case shown="True" w1484 {
              frame False {
              }
              frame True {
                n1043 = property on="Sample Channel\nFlow" class="Bool (strict)"("Val(Sgnl)"=TRUE ("Value (Signaling)")) -> ()  [unwired: 2 in, 2 out]
              }
            }
            n1044 = property on="Got DNA bead" class="Bool"("Key Focus"=FALSE) -> ()  [unwired: 2 in, 2 out]
          }
          frame #1 {
            n1045 = property on="Inject Pump 1" class="Bool (strict)"("Val(Sgnl)"=FALSE ("Value (Signaling)")) -> ()  [unwired: 2 in, 2 out]
          }
          frame #2 {
            n1046 = property on="Cal/Data Acq. Spot" class="Bool (strict)"("Val(Sgnl)"=TRUE ("Value (Signaling)")) -> ()  [unwired: 2 in, 2 out]
          }
        }
      }
      event "Take Stepping Data": Value Change {
        n1047 = event-data() -> ()  [unwired: 1 in, 5 out]
        n1048 = local read "Save ave N"() -> (w1496:dbl)
        n1049 = flat-sequence {
          tunnel: w1496 -> [w1498]
          tunnel: [w1498] -> w1491
          tunnel: [w1500] -> w1492
          tunnel: w1491 -> [w1500]
          tunnel: [w1502] -> w1493
          tunnel: w1492 -> [w1502]
          tunnel: [w1505] -> w1494
          tunnel: w1493 -> [w1505]
          tunnel: [w1507] -> w1495
          tunnel: w1494 -> [w1507]
          tunnel: [w1509] -> w1489
          tunnel: w1495 -> [w1509]
          tunnel: w1489 -> [w1512]
          tunnel: [w1512] -> w1488
          tunnel: w1488 -> [w1513]
          tunnel: [w1513] -> w1490
          tunnel: w1490 -> [w1519]
          frame #0 {
            n1050 = property on="Save ave N" class="DigNum (strict)"("Val(Sgnl)"="Save ave factor") -> ()  [unwired: 2 in, 2 out]
          }
          frame #1 {
            n1051 = Wait (ms)(milliseconds to wait=u32 100) -> ()  [unwired: 1 out]
          }
          frame #2 {
            n1052 = local read "Offset 2 Start (MHz)"() -> (w1504:dbl)
            n1053 = property on="Saved AOD Raster Scan Parameter Sets" class="Arr (strict)"("Index Values"=u32[] [2]) -> ()  [unwired: 2 in, 2 out]
            n1054 = property on="Trap Delta (MHz)" class="DigNum (strict)"("Val(Sgnl)"=w1504) -> ()  [unwired: 2 in, 2 out]
          }
          frame #3 {
            n1055 = property on="Load parameters" class="Bool (strict)"("Val(Sgnl)"=TRUE ("Value (Signaling)")) -> ()  [unwired: 2 in, 2 out]
          }
          frame #4 {
            n1056 = Wait (ms)(milliseconds to wait=u32 100) -> ()  [unwired: 1 out]
          }
          frame #5 {
            n1057 = property on="Trap Raster Scan" class="Bool (strict)"("Val(Sgnl)"=TRUE ("Value (Signaling)")) -> ()  [unwired: 2 in, 2 out]
          }
          frame #6 {
            n1058 = Wait (ms)(milliseconds to wait=u32 1000) -> ()  [unwired: 1 out]
          }
          frame #7 {
            n1059 = while {
              stop <- w1516 stop-if-true
              n1060 = local read "Raster Scanning..."() -> (w1518:bool)
              n1061 = local read "Saving..."() -> (w1517:bool)
              n1062 = Not(x=w1517) -> (.not. x?=w1514:bool)
              n1063 = Not(x=w1518) -> (.not. x?=w1515:bool)
              n1064 = And(x=w1515, y=w1514) -> (x .and. y?=w1516:bool)
            }
          }
          frame #8 {
            n1065 = property on="Save ave N" class="DigNum (strict)"("Val(Sgnl)"=w1519) -> ()  [unwired: 2 in, 2 out]
          }
        }
      }
      event "Step Size (nm)": Value Change {
        n1066 = event-data() -> ()  [unwired: 1 in, 5 out]
        n1067 = flat-sequence {
          frame #0 {
            n1068 = property on="Saved AOD Raster Scan Parameter Sets" class="Arr (strict)"("Index Values"=u32[] [1]) -> ()  [unwired: 2 in, 2 out]
          }
          frame #1 {
            n1069 = Multiply(x="N Steps", y="Step Size (nm)") -> (x*y=w1521:dbl)
            n1070 = property on="Scan Speed AOD (nm/s) 2" class="DigNum (strict)"("Value"="Step Size (nm)") -> ()  [unwired: 2 in, 2 out]
            n1071 = property on="Step Size AOD (nm) 2" class="DigNum (strict)"("Value"="Step Size (nm)") -> ()  [unwired: 2 in, 2 out]
            n1072 = property on="Scan Range AOD (nm) 2" class="DigNum (strict)"("Value"=w1521) -> ()  [unwired: 2 in, 2 out]
          }
        }
      }
      event "Take Detection Laser\nImage": Value Change {
        n1073 = event-data() -> ()  [unwired: 1 in, 5 out]
        n1074 = flat-sequence {
          tunnel: [w1549] -> w1539
          tunnel: [w1548] -> w1532
          tunnel: [w1547] -> w1524
          tunnel: [w1552] -> w1540
          tunnel: w1539 -> [w1552]
          tunnel: [w1551] -> w1533
          tunnel: w1532 -> [w1551]
          tunnel: [w1550] -> w1525
          tunnel: w1524 -> [w1550]
          tunnel: [w1556] -> w1541
          tunnel: w1540 -> [w1556]
          tunnel: [w1555] -> w1534
          tunnel: w1533 -> [w1555]
          tunnel: [w1554] -> w1526
          tunnel: w1525 -> [w1554]
          tunnel: [w1562] -> w1542
          tunnel: w1541 -> [w1562]
          tunnel: [w1561] -> w1535
          tunnel: w1534 -> [w1561]
          tunnel: [w1560] -> w1527
          tunnel: w1526 -> [w1560]
          tunnel: [w1566] -> w1543
          tunnel: w1542 -> [w1566]
          tunnel: [w1565] -> w1536
          tunnel: w1535 -> [w1565]
          tunnel: [w1564] -> w1528
          tunnel: w1527 -> [w1564]
          tunnel: [w1570] -> w1544
          tunnel: w1543 -> [w1570]
          tunnel: [w1569] -> w1537
          tunnel: w1536 -> [w1569]
          tunnel: [w1568] -> w1529
          tunnel: w1528 -> [w1568]
          tunnel: [w1574] -> w1545
          tunnel: w1544 -> [w1574]
          tunnel: [w1573] -> w1538
          tunnel: w1537 -> [w1573]
          tunnel: [w1572] -> w1530
          tunnel: w1529 -> [w1572]
          tunnel: w1545 -> [w1580]
          tunnel: w1538 -> [w1579]
          tunnel: [w1577] -> w1531
          tunnel: w1530 -> [w1577]
          tunnel: w1531 -> [w1581]
          frame #0 {
            n1075 = local read "Laser interlacing mode"() -> (w1548:enum32{"Laser ON", "Laser OFF", "Interlace"})
            n1076 = local read "Green FB On/Off"() -> (w1547:bool)
            n1077 = local read "Green Laser ON"() -> (w1549:bool)
          }
          frame #1 {
            n1078 = property on="Green FB On/Off" class="Bool (strict)"("Val(Sgnl)"=FALSE ("Value (Signaling)")) -> ()  [unwired: 2 in, 2 out]
          }
          frame #2 {
            n1079 = property on="Green Laser ON" class="Bool (strict)"("Val(Sgnl)"=TRUE ("Value (Signaling)")) -> ()  [unwired: 2 in, 2 out]
            n1080 = property on="Flip Green Filter" class="Bool (strict)"("Val(Sgnl)"=TRUE ("Value (Signaling)")) -> ()  [unwired: 2 in, 2 out]
            n1081 = property on="Laser interlacing mode" class="RadioBtnsControl (strict)"("Val(Sgnl)"=enum32{"Laser ON", "Laser OFF", "Interlace"}."Laser ON" ("Value (Signaling)")) -> ()  [unwired: 2 in, 2 out]
          }
          frame #3 {
            n1082 = Wait (ms)(milliseconds to wait=u32 500) -> ()  [unwired: 1 out]
          }
          frame #4 {
            n1083 = property on="Confocal Image" class="Bool (strict)"("Val(Sgnl)"=TRUE ("Value (Signaling)")) -> ()  [unwired: 2 in, 2 out]
          }
          frame #5 {
            n1084 = Wait (ms)(milliseconds to wait=u32 2000) -> ()  [unwired: 1 out]
          }
          frame #6 {
            n1085 = while {
              stop <- w1575 stop-if-true
              n1086 = local read "Saving..."() -> (w1576:bool)
              n1087 = Not(x=w1576) -> (.not. x?=w1575:bool)
            }
          }
          frame #7 {
            n1088 = property on="Flip Green Filter" class="Bool (strict)"("Val(Sgnl)"=TRUE ("Value (Signaling)")) -> ()  [unwired: 2 in, 2 out]
            n1089 = property on="Green Laser ON" class="Bool (strict)"("Val(Sgnl)"=w1580) -> ()  [unwired: 2 in, 2 out]
            n1090 = property on="Laser interlacing mode" class="RadioBtnsControl (strict)"("Val(Sgnl)"=w1579) -> ()  [unwired: 2 in, 2 out]
          }
          frame #8 {
            n1091 = property on="Green FB On/Off" class="Bool (strict)"("Val(Sgnl)"=w1581) -> ()  [unwired: 2 in, 2 out]
          }
        }
      }
      event "Stop All": Value Change {
        n1092 = event-data() -> ()  [unwired: 1 in, 5 out]
        n1093 = local read "Stop All"() -> (w1582:bool)
      }
    }
    n1094 = node-c288() -> ()  [unwired: 1 in, 1 out]
  }
  n1095 = timed-loop "Basic control parameters (all FPGA settings, other basic controls)" {
    tunnel: w8 -> [w1591]
    shift-right: [w1590] -> _
    shift-left: errorcluster {"status"=FALSE, "code"=0, "source"=""} ("error out") -> [w1589]
    tunnel: [w1588] -> _
    timing: w122 -> [_]
    timing-out: [_] -> w121
    tunnel: w95 -> [w1587]
    tunnel: w67 -> [w1586]
    tunnel: w66 -> [w1585]
    tunnel: w65 -> [w1584]
    tunnel: w64 -> [w1583]
    stop <- w1588 stop-if-true
    n1096 = node-c288() -> ()  [unwired: 2 out]
    n1097 = event shown="[21] \"Invert laser interlacing\": Value Change" {
      selector: _ -> [_ _ _ _ _ _ _ _ _ _ _ _ _ _ _ _ _ _ _ _ _ _ _ _ _ _ _ _ _ _ _ _ _ _ _ _ _ _ _ _ _ _ _ _ _ _ _ _ _ _ _ _ _ _ _ _ _ _ _ _ _ _ _ _ _ _ _ _ _ _ _ _ _ _]
      dyn-events: _ -> [_ _ _ _ _ _ _ _ _ _ _ _ _ _ _ _ _ _ _ _ _ _ _ _ _ _ _ _ _ _ _ _ _ _ _ _ _ _ _ _ _ _ _ _ _ _ _ _ _ _ _ _ _ _ _ _ _ _ _ _ _ _ _ _ _ _ _ _ _ _ _ _ _ _]
      timeout: _ -> [_ _ _ _ _ _ _ _ _ _ _ _ _ _ _ _ _ _ _ _ _ _ _ _ _ _ _ _ _ _ _ _ _ _ _ _ _ _ _ _ _ _ _ _ _ _ _ _ _ _ _ _ _ _ _ _ _ _ _ _ _ _ _ _ _ _ _ _ _ _ _ _ _ _]
      tunnel: w1591 -> [w1632 _ _ _ w1670 _ w1692 _ _ _ _ w1758 _ _ w1801 w1807 w1814 w1819 w1910 _ w1926 w1951 w1972 w1993 w2014 w2043 w2069 w2072 w2076 w2171 w2176 w2214 _ w2249 w2253 w2264 w2268 w2272 _ w2280 _ _ _ _ _ _ _ _ _ _ _ _ _ _ _ _ _ w2658 _ w2675 _ w2682 w2700 _ w2707 w2715 w2730 w2746 w2752 _ w2761 _ w2780 _]
      tunnel: [w1631 _ _ _ w1660 _ w1691 _ _ w1723 _ w1737 _ _ w1800 w1803 w1813 w1816 w1904 _ w1925 w1950 w1970 w1991 w2012 w2037 w2067 _ w2074 w2169 w2174 w2212 _ w2247 w2251 w2255 w2266 w2270 _ w2278 _ _ _ _ _ _ _ _ _ _ _ _ _ _ _ _ _ w2656 _ _ _ _ w2697 _ _ _ _ _ _ _ _ _ _ _] -> w1590
      tunnel: w1589 -> [w1630 _ _ _ w1669 _ w1690 _ _ w1723 _ w1757 _ _ w1799 w1802 w1812 w1815 w1909 _ w1924 w1949 w1971 w1992 w2013 w2042 w2068 w2071 w2075 w2170 w2175 w2213 _ w2248 w2252 w2263 w2267 w2271 _ w2279 _ _ _ _ _ _ _ _ _ _ _ _ _ _ _ _ _ w2657 _ w2674 _ w2681 w2699 _ w2706 w2714 w2729 w2745 w2751 _ w2760 _ w2779 _]